vi "HFRR ADV v039 new software.vi"() -> ()   [LabVIEW 2025] (continued)
            n257 = Format Into String(format string="%<%I_%M_%S_%p_%d_%B_%Y>T", w342) -> (resulting string=w341:string)  [unwired: 2 in, 1 out]
            n258 = local write "FILE"(w341) -> ()
          }
        }
        n259 = local read "Auto"() -> (w339:bool)
        n260 = Not(x=w339) -> (.not. x?=w338:bool)
        n261 = local write "Auto"(w338) -> ()
      }
      event "Auto Start Temp": Value Change {
        n262 = event-data() -> ()  [unwired: 1 in, 6 out]
        n263 = local read "Auto Start Test"() -> (w345:bool)
        n264 = case shown="True" w345 {
          frame False {
            n265 = stacked-sequence {
              frame #0 {
                n266 = local write "START TEMP"(FALSE ("START TEMP")) -> ()
              }
              frame #1 {
                n267 = Wait (ms)(milliseconds to wait=u32 2000) -> ()  [unwired: 1 out]
              }
              frame #2 {
                n268 = local write "Due Write"("VC;0") -> ()
              }
              frame #3 {
                n269 = Wait (ms)(milliseconds to wait=u32 2000) -> ()  [unwired: 1 out]
              }
              frame #4 {
                w355 = T19."Enabled" ("Disabled")
                (unwired) T26."Imaging" ("Main Dashboard Buttons")
                w356 = "" ("FILE")
                n270 = local write "Main Tab"(T2."Adv Scar" ("Main Tab")) -> ()
                n271 = local write "measured_stroke"(0.0 ("measured_stroke")) -> ()
                n272 = local write "Main Dashboard Buttons"(T1."Imaging" ("Main Dashboard Buttons")) -> ()
                n273 = property on="RUN" class="Bool (strict)"("Visible"=TRUE) -> ()  [unwired: 2 in, 2 out]
                n274 = local write "Due Write"("VC;0") -> ()
                n275 = local write "TEST FILE NAM,E SAVED"(FALSE ("TEST FILE NAM,E SAVED")) -> ()
                n276 = local write "Fuel Discription :"(w356) -> ()
                n277 = local write "Batch Ref Num :"(w356) -> ()
                n278 = local write "Remarks :"(w356) -> ()
                n279 = local write "FILE"(w356) -> ()
                n280 = property on="FRICVALZ 4" class="Bool (strict)"("DisabledEnum"=w355) -> ()  [unwired: 2 in, 2 out]
                n281 = property on="FRICVALZ 2" class="Bool (strict)"("DisabledEnum"=w355) -> ()  [unwired: 2 in, 2 out]
                n282 = property on="FRICVALZ 3" class="Bool (strict)"("DisabledEnum"=w355) -> ()  [unwired: 2 in, 2 out]
              }
            }
          }
          frame True {
            n283 = stacked-sequence {
              frame #0 {
                n284 = local write "Due Write"("DAC;200") -> ()
              }
              frame #1 {
                n285 = Wait (ms)(milliseconds to wait=u32 1500) -> ()  [unwired: 1 out]
              }
              frame #2 {
                n286 = local write "Due Write"("DAC;200") -> ()
              }
              frame #3 {
                n287 = Wait (ms)(milliseconds to wait=u32 1000) -> ()  [unwired: 1 out]
              }
              frame #4 {
                n288 = local write "Due Write"("VC;1") -> ()
              }
              frame #5 {
                n289 = Wait (ms)(milliseconds to wait=u32 2000) -> ()  [unwired: 1 out]
              }
              frame #6 {
                n290 = local write "Due Write"("VC;1") -> ()
              }
              frame #7 {
                n291 = Wait (ms)(milliseconds to wait=u32 2000) -> ()  [unwired: 1 out]
              }
              frame #8 {
                w367 = T19."Disabled" ("Disabled")
                n292 = property on="RUN" class="Bool (strict)"("Visible"=FALSE) -> ()  [unwired: 2 in, 2 out]
                n293 = property on="FRICVALZ 4" class="Bool (strict)"("DisabledEnum"=w367) -> ()  [unwired: 2 in, 2 out]
                n294 = property on="FRICVALZ 2" class="Bool (strict)"("DisabledEnum"=w367) -> ()  [unwired: 2 in, 2 out]
                n295 = property on="FRICVALZ 3" class="Bool (strict)"("DisabledEnum"=w367) -> ()  [unwired: 2 in, 2 out]
                "START TEMP" <- TRUE
              }
            }
          }
        }
      }
      event "FILE", "USERNAME", "USER ID": Mouse Enter {
        n296 = event-data() -> ()  [unwired: 1 in, 4 out]
        n297 = dll-call lib="kernel32.dll" fn="Wow64DisableWow64FsRedirection"("OldValue"=0) -> (error out=w374:errorcluster, "OldValue"=w372:i32)  [unwired: 4 in, 1 out]
        n298 = call <vilib>:"System Exec.vi"("run minimized? (F)"=TRUE, "error in (no error)"=w374, "command line"="C:\\Program Files\\Common Files\\Microsoft Shared\\Ink\\TabTip.exe") -> ("error out"=w373:errorcluster)  [unwired: 5 in, 3 out]
        n299 = dll-call lib="kernel32.dll" fn="Wow64EnableWow64FsRedirection"(error in=w373, "OldValue"=w372) -> ()  [unwired: 4 in, 2 out]
      }
      event "EDIT": Value Change {
        n300 = event-data() -> ()  [unwired: 1 in, 6 out]
        n301 = local read "EDIT"() -> (w375:bool)
        n302 = case shown="False" w375 {
          frame False {
            n303 = control-ref of="This VI"() -> (w392:refnum<vi>)
            n304 = property class="VI"(reference=w392) -> (reference out=w383:refnum<vi>, error out=w387:errorcluster, "Panel"=w391:refnum<vi>)  [unwired: 1 in]
            n305 = property class="Pnl"(reference=w391, error in=w387) -> (reference out=w385:refnum<vi>, error out=w388:errorcluster, "Panes[]"=w390:refnum<vi>[])
            n306 = for {
              tunnel: w390 -> [w398] mode=indexing
              tunnel: T24."Always Off" ("Horizontal Scrollbar Visibility") -> [w397]
              tunnel: w388 -> [w394]
              tunnel: [w393] -> w386
              n307 = property class="Pane"(reference=w398, error in=w394, "HorizScrollbarVisibility"=w397) -> (reference out=w395:refnum<vi>, error out=w396:errorcluster)
              n308 = Close Reference(reference=w395, error in (no error)=w396) -> (error out=w393:errorcluster)
            }
            n309 = Close Reference(reference=w385, error in (no error)=w386) -> (error out=w384:errorcluster)
            n310 = Close Reference(reference=w383, error in (no error)=w384) -> (error out=w378:errorcluster)
            "error out 7" <- w378
            n311 = call <vilib>:"Clear Errors.vi"("error in (no error)"=w378) -> ("error out"=w377:errorcluster)  [unwired: 5 in, 1 out]
            n312 = local write "Service Password enable"(FALSE ("Service Password enable")) -> ()
            n313 = call <userlib>:"Fit VI window to Largest Dec.vi"("error in (no error)"=w377, "border spacing (2 px)"=1) -> ("error out"=w382:errorcluster, "dup VI Ref"=w380:refnum<vi>)  [unwired: 4 in]
            n314 = invoke on="Invoke Node" class="VI" method="FP.Run-Time Position.Maximized"(reference=w380, error in=w382) -> (error out=w381:errorcluster)  [unwired: 2 in, 3 out]
            n315 = call <vilib>:"Clear Errors.vi"("error in (no error)"=w381) -> ()  [unwired: 5 in, 2 out]
          }
          frame True {
          }
        }
      }
      event "Heater Button": Value Change {
        n316 = event-data() -> ()  [unwired: 1 in, 6 out]
        n317 = local read "Heater Button"() -> (w399:bool)
        n318 = case shown="True" w399 {
          frame True {
            n319 = stacked-sequence {
              frame #0 {
                n320 = Wait (ms)(milliseconds to wait=u32 1500) -> ()  [unwired: 1 out]
              }
              frame #1 {
                n321 = local read "Set Temp"() -> (w401:dbl)
                n322 = Number To Fractional String(number=w401, precision (6)=i16 2) -> (F-format string=w404:string)  [unwired: 2 in]
                n323 = Concatenate Strings("ST;" ("Command"), w404) -> (w403:string)
                n324 = local write "Due Write"(w403) -> ()
              }
              frame #2 {
                n325 = Wait (ms)(milliseconds to wait=u32 1500) -> ()  [unwired: 1 out]
              }
              frame #3 {
                n326 = local write "Due Write"("HE;1" ("Command")) -> ()
              }
              frame #4 {
                n327 = Wait (ms)(milliseconds to wait=u32 1500) -> ()  [unwired: 1 out]
              }
              frame #5 {
                n328 = stacked-sequence {
                  frame #0 {
                    n329 = Wait (ms)(milliseconds to wait=u32 1500) -> ()  [unwired: 1 out]
                  }
                  frame #1 {
                    n330 = local read "Set Temp"() -> (w410:dbl)
                    n331 = Number To Fractional String(number=w410, precision (6)=i16 2) -> (F-format string=w413:string)  [unwired: 2 in]
                    n332 = Concatenate Strings("ST;" ("Command"), w413) -> (w412:string)
                    n333 = local write "Due Write"(w412) -> ()
                  }
                  frame #2 {
                    n334 = Wait (ms)(milliseconds to wait=u32 1500) -> ()  [unwired: 1 out]
                  }
                  frame #3 {
                    n335 = local write "Due Write"("HE;1" ("Command")) -> ()
                  }
                  frame #4 {
                    n336 = Wait (ms)(milliseconds to wait=u32 1500) -> ()  [unwired: 1 out]
                  }
                }
              }
            }
          }
          frame False {
            n337 = stacked-sequence {
              frame #0 {
                n338 = Wait (ms)(milliseconds to wait=u32 1500) -> ()  [unwired: 1 out]
              }
              frame #1 {
                n339 = Concatenate Strings("ST;" ("Command"), "0" ("string")) -> (w420:string)
                n340 = local write "Due Write"(w420) -> ()
              }
              frame #2 {
                n341 = Wait (ms)(milliseconds to wait=u32 1500) -> ()  [unwired: 1 out]
              }
              frame #3 {
                n342 = local write "Due Write"("HE;0" ("Command")) -> ()
              }
              frame #4 {
                n343 = Wait (ms)(milliseconds to wait=u32 1500) -> ()  [unwired: 1 out]
              }
            }
          }
        }
      }
      event "Headen Service Button": Value Change {
        n344 = event-data() -> ()  [unwired: 1 in, 6 out]
        n345 = local read "Headen Service Button"() -> (w425:bool)
        n346 = case shown="True" w425 {
          frame False {
            n347 = property on="Password 3" class="Clust (strict)"("Visible"=FALSE) -> ()  [unwired: 2 in, 2 out]
            n348 = property on="Service Password Log" class="Str"("Visible"=FALSE) -> ()  [unwired: 2 in, 2 out]
          }
          frame True {
            n349 = property on="Password 3" class="Clust (strict)"("Visible"=TRUE) -> ()  [unwired: 2 in, 2 out]
            n350 = property on="Service Password Log" class="Str"("Visible"=TRUE) -> ()  [unwired: 2 in, 2 out]
          }
        }
      }
      event "Password 3.Service Password": Value Change {
        n351 = event-data() -> ()  [unwired: 1 in, 6 out]
        n352 = Unbundle By Name("Password 3") -> ("Service Password"=w432:string)
        n353 = call <vilib>:"Trim Whitespace.vi"("string"=w432) -> ("trimmed string"=w430:string)  [unwired: 1 in]
        n354 = Equal?(x=w430, y="Service@123") -> (x = y?=w431:bool)
        n355 = case shown="False" w431 {
          selector: w431 -> [w435 w437]
          frame False {
            n356 = local write "Service Password enable"(w435) -> ()
            n357 = property on="Service Password Log" class="Str"("Visible"=TRUE) -> ()  [unwired: 2 in, 2 out]
          }
          frame True {
            n358 = property on="Service Password Log" class="Str"("Visible"=FALSE) -> ()  [unwired: 2 in, 2 out]
            "Service Password enable" <- w437
          }
        }
      }
      event "Sign In": Value Change {
        w439 = FALSE ("Visible")
        n359 = event-data() -> ()  [unwired: 1 in, 6 out]
        n360 = property on="About" class="Clust (strict)"("Visible"=w439) -> ()  [unwired: 2 in, 2 out]
        n361 = property on="Password 3" class="Clust (strict)"("Visible"=w439) -> ()  [unwired: 2 in, 2 out]
        n362 = property on="Service Password Log" class="Str"("Visible"=FALSE) -> ()  [unwired: 2 in, 2 out]
      }
      event "Info": Value Change {
        n363 = event-data() -> ()  [unwired: 1 in, 6 out]
        n364 = local read "Info"() -> (w441:bool)
        n365 = case shown="False" w441 {
          frame False {
            n366 = property on="About" class="Clust (strict)"("Visible"=FALSE) -> ()  [unwired: 2 in, 2 out]
          }
          frame True {
            n367 = property on="About" class="Clust (strict)"("Visible"=TRUE) -> ()  [unwired: 2 in, 2 out]
          }
        }
      }
      event "Calibration": Value Change {
        n368 = event-data() -> ()  [unwired: 1 in, 6 out]
        n369 = local read "Calibration"() -> (w445:bool)
        n370 = case shown="False" w445 {
          frame False {
            n371 = local write "Cal Password"("" ("Cal Password")) -> ()
            n372 = property on="Calibration 2" class="TabCtl (strict)"("Visible"=FALSE) -> ()  [unwired: 2 in, 2 out]
          }
          frame True {
            n373 = property on="Calibration 2" class="TabCtl (strict)"("Visible"=TRUE) -> ()  [unwired: 2 in, 2 out]
            n374 = local write "Cal Password"("" ("Cal Password")) -> ()
          }
        }
        n375 = property on="Wrong Password" class="Str"("Visible"=FALSE) -> ()  [unwired: 2 in, 2 out]
      }
      event "Cal Password": Value Change {
        n376 = event-data() -> ()  [unwired: 1 in, 6 out]
        n377 = local read "Cal Password"() -> (w453:string)
        n378 = call <vilib>:"Trim Whitespace.vi"("string"=w453) -> ("trimmed string"=w452:string)  [unwired: 1 in]
        n379 = Equal?(x=w452, y="Cal@321") -> (x = y?=w450:bool)
        n380 = case shown="True" w450 {
          frame False {
            n381 = property on="Wrong Password" class="Str"("Visible"=TRUE) -> ()  [unwired: 2 in, 2 out]
          }
          frame True {
            n382 = property on="Wrong Password" class="Str"("Visible"=FALSE) -> ()  [unwired: 2 in, 2 out]
            n383 = local write "Main Tab"(T2."About" ("Main Tab")) -> ()
            n384 = local write "Cal Password"("" ("Cal Password")) -> ()
            n385 = local write "Main Dashboard Buttons"(T1."About" ("Main Dashboard Buttons")) -> ()
            n386 = property on="Calibration 2" class="TabCtl (strict)"("Visible"=FALSE) -> ()  [unwired: 2 in, 2 out]
            n387 = local write "Calibration"(FALSE ("Calibration")) -> ()
          }
        }
      }
      event "Calibration Selection": Value Change {
        n388 = event-data() -> ()  [unwired: 1 in, 6 out]
        n389 = local read "Calibration Selection"() -> (w462:T8)
        n390 = case shown="\"Stroke Calibration\"" w462 {
          tunnel: [T7."Stroke" ("Main Calibration Tab") T7."Friction" ("Main Calibration Tab") T7."Main" ("Main Calibration Tab") T7."Temperature" ("Main Calibration Tab")] -> w461
          frame "Stroke Calibration" {
          }
          frame "Friction Force Calibration" {
          }
          frame Default {
          }
          frame "Temperature Calibration" {
          }
        }
        n391 = local write "Main Calibration Tab"(w461) -> ()
      }
      event "Back Stroke": Value Change {
        n392 = event-data() -> ()  [unwired: 1 in, 6 out]
        n393 = local write "Main Stroke Tab"(T9."Step 1" ("Main Stroke Tab")) -> ()
        n394 = local write "Main Calibration Tab"(T7."Main" ("Main Calibration Tab")) -> ()
        n395 = local write "Back Stroke"(FALSE ("Back Stroke")) -> ()
      }
      event "Step 2 Back": Value Change {
        n396 = event-data() -> ()  [unwired: 1 in, 6 out]
        n397 = local write "Main Stroke Tab"(T9."Step 1" ("Main Stroke Tab")) -> ()
        n398 = local write "Step 2 Back"(FALSE ("Back Stroke")) -> ()
      }
      event "Step 3 Back": Value Change {
        n399 = event-data() -> ()  [unwired: 1 in, 6 out]
        n400 = local write "Main Stroke Tab"(T9."Step 2" ("Main Stroke Tab")) -> ()
        n401 = local write "Step 3 Back"(FALSE ("Back Stroke")) -> ()
      }
      event "Step 4 Back": Value Change {
        n402 = event-data() -> ()  [unwired: 1 in, 6 out]
        n403 = local write "Main Stroke Tab"(T9."Step 3" ("Main Stroke Tab")) -> ()
        n404 = local write "Step 4 Back"(FALSE ("Back Stroke")) -> ()
      }
      event "Step 5 Back": Value Change {
        n405 = event-data() -> ()  [unwired: 1 in, 6 out]
        n406 = local write "Main Stroke Tab"(T9."Step 4" ("Main Stroke Tab")) -> ()
        n407 = local write "Step 5 Back"(FALSE ("Back Stroke")) -> ()
      }
      event "Step 6 Back": Value Change {
        n408 = event-data() -> ()  [unwired: 1 in, 6 out]
        n409 = local write "Main Stroke Tab"(T9."Step 5" ("Main Stroke Tab")) -> ()
        n410 = local write "Step 6 Back"(FALSE ("Back Stroke")) -> ()
      }
      event "Back Stroke step 7": Value Change {
        n411 = event-data() -> ()  [unwired: 1 in, 6 out]
        n412 = local write "Main Stroke Tab"(T9."Step 5" ("Main Stroke Tab")) -> ()
        n413 = local write "Back Stroke step 7"(FALSE ("Back Stroke")) -> ()
      }
      event "Back Stroke step 8": Value Change {
        n414 = event-data() -> ()  [unwired: 1 in, 6 out]
        n415 = local write "Main Stroke Tab"(T9."Step 7" ("Main Stroke Tab")) -> ()
        n416 = local write "Back Stroke step 8"(FALSE ("Back Stroke")) -> ()
      }
      event "Back Stroke 8": Value Change {
        n417 = event-data() -> ()  [unwired: 1 in, 6 out]
        n418 = local write "MOVE CARRIAGE TO"(0.2 ("MOVE CARRIAGE TO")) -> ()
        n419 = local write "Main Stroke Tab"(T9."Step 1" ("Main Stroke Tab")) -> ()
        n420 = local write "Back Stroke 8"(FALSE ("Back Stroke 8")) -> ()
      }
      event "Continue Stroke": Value Change {
        n421 = event-data() -> ()  [unwired: 1 in, 6 out]
        n422 = local write "Main Stroke Tab"(T9."Step 2" ("Main Stroke Tab")) -> ()
        n423 = local write "Continue Stroke"(FALSE ("Continue Stroke")) -> ()
      }
      event "Continue Stroke step 2": Value Change {
        n424 = event-data() -> ()  [unwired: 1 in, 6 out]
        n425 = local write "Main Stroke Tab"(T9."Step 3" ("Main Stroke Tab")) -> ()
        n426 = local write "Continue Stroke step 2"(FALSE ("Continue Stroke")) -> ()
      }
      event "Continue Stroke step 3": Value Change {
        n427 = event-data() -> ()  [unwired: 1 in, 6 out]
        n428 = local write "Main Stroke Tab"(T9."Step 4" ("Main Stroke Tab")) -> ()
        n429 = local write "Continue Stroke step 3"(FALSE ("Continue Stroke")) -> ()
      }
      event "Continue Stroke step 4": Value Change {
        n430 = event-data() -> ()  [unwired: 1 in, 6 out]
        n431 = local write "Main Stroke Tab"(T9."Step 5" ("Main Stroke Tab")) -> ()
        n432 = local write "Continue Stroke step 4"(FALSE ("Continue Stroke")) -> ()
      }
      event "Continue Stroke step 5": Value Change {
        n433 = event-data() -> ()  [unwired: 1 in, 6 out]
        n434 = local write "Main Stroke Tab"(T9."Step 7" ("Main Stroke Tab")) -> ()
        n435 = local write "Continue Stroke step 5"(FALSE ("Continue Stroke")) -> ()
      }
      event "Continue Stroke step 6": Value Change {
        n436 = event-data() -> ()  [unwired: 1 in, 6 out]
        n437 = local write "Main Stroke Tab"(T9."Step 7" ("Main Stroke Tab")) -> ()
        n438 = local write "Continue Stroke step 6"(FALSE ("Continue Stroke")) -> ()
      }
      event "Continue Stroke step 7": Value Change {
        w501 = FALSE ("0.2mm")
        n439 = event-data() -> ()  [unwired: 1 in, 6 out]
        n440 = local write "1.2"(w501) -> ()
        n441 = local write "1.0 2"(w501) -> ()
        n442 = local write "0.8 2"(w501) -> ()
        n443 = local write "0.6 2"(w501) -> ()
        n444 = local write "0.4 2"(w501) -> ()
        n445 = local write "0.2 2"(w501) -> ()
        n446 = local write "1.2 mm"(w501) -> ()
        n447 = local write "1.0 mm"(w501) -> ()
        n448 = local write "0.6 mm"(w501) -> ()
        n449 = local write "0.4 mm"(w501) -> ()
        n450 = local write "0.8mm"(w501) -> ()
        n451 = local write "0.2mm"(w501) -> ()
        n452 = local write "Main Stroke Tab"(T9."Step 8" ("Main Stroke Tab")) -> ()
        n453 = local write "Continue Stroke step 7"(FALSE ("Continue Stroke")) -> ()
        n454 = local write "Stroke Test Complete"(T10."Test Progress" ("Stroke Test Complete")) -> ()
        "Position Measurment Temp" <- 4.0 ("Position Measurment Temp")
        "Calibration Tare" <- TRUE ("Calibration Tare")
        "MOVE CARRIAGE TO" <- 1.0 ("MOVE CARRIAGE TO")
      }
      event "Continue Stroke step 8": Value Change {
        n455 = event-data() -> ()  [unwired: 1 in, 6 out]
        n456 = local read "LVDT STROKE  Calibration"() -> (w506:dbl)
        n457 = local read "Position Measurment Temp"() -> (w507:dbl)
        n458 = case shown="7" w507 {
          selector: w507 -> [_ w512 w520 w525 _ w533 w536 w537]
          tunnel: w506 -> [w509 w513 w516 w521 w527 w530 _ _]
          frame 0, Default {
            w511 = TRUE ("0.2mm")
            n459 = local write "Position Measurment Temp"(4.0 ("Position Measurment Temp")) -> ()
            n460 = local write "0.2mm"(w511) -> ()
            n461 = local write "0.2 2"(w511) -> ()
            n462 = local write "MOVE CARRIAGE TO"(1.0 ("MOVE CARRIAGE TO")) -> ()
            "Calibration 0.2" <- w509
          }
          frame 1 {
            w515 = TRUE ("0.4 mm")
            n463 = local write "Calibration 0.4"(w513) -> ()
            n464 = local write "Position Measurment Temp"(w512) -> ()
            n465 = local write "0.4 mm"(w515) -> ()
            n466 = local write "MOVE CARRIAGE TO"(0.6 ("MOVE CARRIAGE TO")) -> ()
            n467 = local write "0.4 2"(w515) -> ()
          }
          frame 2 {
            w518 = TRUE ("0.6 mm")
            n468 = Increment(x=w520) -> (x+1=w519:i32)
            n469 = local write "Calibration 0.6"(w516) -> ()
            n470 = local write "Position Measurment Temp"(w519) -> ()
            n471 = local write "0.6 2"(w518) -> ()
            n472 = local write "0.6 mm"(w518) -> ()
            n473 = local write "MOVE CARRIAGE TO"(0.8 ("MOVE CARRIAGE TO")) -> ()
          }
          frame 3 {
            w522 = TRUE ("0.6 mm")
            n474 = Increment(x=w525) -> (x+1=w524:i32)
            n475 = local write "Position Measurment Temp"(w524) -> ()
            n476 = local write "MOVE CARRIAGE TO"(1.0 ("MOVE CARRIAGE TO")) -> ()
            n477 = local write "0.8mm"(w522) -> ()
            n478 = local write "0.8 2"(w522) -> ()
            "Calibration 0.8" <- w521
          }
          frame 4 {
            w528 = TRUE ("0.6 mm")
            n479 = local write "Position Measurment Temp"(6.0 ("Position Measurment Temp")) -> ()
            n480 = local write "MOVE CARRIAGE TO"(1.0 ("MOVE CARRIAGE TO")) -> ()
            n481 = local write "1.0 mm"(w528) -> ()
            n482 = local write "1.0 2"(w528) -> ()
            "Calibration 1.0" <- w527
          }
          frame 5 {
            w531 = TRUE ("0.6 mm")
            n483 = Increment(x=w533) -> (x+1=w532:i32)
            n484 = local write "Position Measurment Temp"(w532) -> ()
            n485 = local write "1.2 mm"(w531) -> ()
            n486 = local write "1.2"(w531) -> ()
            "Calibration 1.2" <- w530
          }
          frame 6 {
            n487 = Increment(x=w536) -> (x+1=w535:i32)
            n488 = local write "Position Measurment Temp"(w535) -> ()
            n489 = local write "Stroke Test Complete"(T10."Stroke Points Completed" ("Stroke Test Complete")) -> ()
          }
          frame 7 {
            n490 = stacked-sequence {
              tunnel: w537 -> [w538 _ _]
              frame #0 {
                n491 = Increment(x=w538) -> (x+1=w539:i32)
                n492 = local write "Main Stroke Tab"(T9."Step 9" ("Main Stroke Tab")) -> ()
                n493 = local write "Position Measurment Temp"(w539) -> ()
                n494 = Insert Into Array(array=dbl[] [], new element #1=0.2 ("new element/subarray"), new element #2=0.4 ("new element/subarray"), new element #3=0.6 ("new element/subarray"), new element #4=0.8 ("new element/subarray"), new element #5=1.0 ("new element/subarray"), new element #6=1.2 ("new element/subarray")) -> (→"1D stroke":dbl[])  [unwired: 1 in]
                n495 = local read "Calibration 1.2"() -> (w541:dbl)
                n496 = local read "Calibration 1.0"() -> (w542:dbl)
                n497 = local read "Calibration 0.8"() -> (w543:dbl)
                n498 = local read "Calibration 0.6"() -> (w544:dbl)
                n499 = local read "Calibration 0.4"() -> (w545:dbl)
                n500 = local read "Calibration 0.2"() -> (w546:dbl)
                n501 = Insert Into Array(array=dbl[] [], new element #1=w546, new element #2=w545, new element #3=w544, new element #4=w543, new element #5=w542, new element #6=w541) -> (→"Calibrated Voltage Value":dbl[])  [unwired: 1 in]
              }
              frame #1 {
                n502 = local read "calibration values"() -> (w569:dbl[])
                n503 = local read "Calibrated Voltage Value"() -> (w571:dbl[])
                n504 = Index Array(array=w569, index #1=1 ("index"), index #2=3 ("index"), index #3=5 ("index"), index #4=7 ("index"), index #5=9 ("index"), index #6=11 ("index")) -> (element #1=w562:dbl, element #2=w561:dbl, element #3=w560:dbl, element #4=w559:dbl, element #5=w558:dbl, element #6=w557:dbl)
                n505 = local read "1D stroke"() -> (w572:dbl[])
                n506 = for {
                  tunnel: [w581] -> w570 mode=indexing
                  tunnel: w572 -> [w580] mode=indexing
                  tunnel: w571 -> [w579] mode=indexing
                  tunnel: w562 -> [w578]
                  tunnel: w561 -> [w577]
                  tunnel: w560 -> [w576]
                  tunnel: w559 -> [w575]
                  tunnel: w558 -> [w574]
                  tunnel: w557 -> [w573]
                  n507 = formula code="if (stroke == 0.2)\n{\n    if ((voltage >= REF_02 - 0.2) && (voltage <= REF_02 + 0.2))\n        status = 1;\n    else\n        status = 0;\n}\nelse if (stroke == 0.4)\n{\n    if ((voltage >= REF_04 - 0.2) && (voltage <= REF_04 + 0.2))\n        status = 1;\n    else\n        status = 0;\n}\nelse if (stroke == 0.6)\n{\n    if ((voltage >= REF_06 - 0.2) && (voltage <= REF_06 + 0.2))\n        status = 1;\n    else\n        status = 0;\n}\nelse if (stroke == 0.8)\n{\n    if ((voltage >= REF_08 - 0.2) && (voltage <= REF_08 + 0.2))\n        status = 1;\n    else\n        status = 0;\n}\nelse if (stroke == 1.0)\n{\n    if ((voltage >= REF_10 - 0.6) && (voltage <= REF_10 + 0.6))\n        status = 1;\n    else\n        status = 0;\n}\nelse if (stroke == 1.2)\n{\n    if ((voltage >= REF_12 - 0.2) && (voltage <= REF_12 + 0.2))\n        status = 1;\n    else\n        status = 0;\n}\nelse\n{\n    status = 0;\n}"("stroke"=w580, "voltage"=w579, "REF_02"=w578, "REF_04"=w577, "REF_06"=w576, "REF_08"=w575, "REF_10"=w574, "REF_12"=w573) -> ("status"=w581:dbl)
                }
                "Status" <- w570
              }
              frame #2 {
                w588 = 1.0
                n508 = local read "Status"() -> (w595:dbl[])
                n509 = Index Array(array=w595) -> (element #1=w594:dbl, element #2=w593:dbl, element #3=w592:dbl, element #4=w591:dbl, element #5=w590:dbl, element #6=w589:dbl)  [unwired: 6 in]
                n510 = Equal?(x=w589, y=w588) -> (x = y?=w582:bool)
                n511 = Equal?(x=w590, y=w588) -> (x = y?=w583:bool)
                n512 = Equal?(x=w591, y=w588) -> (x = y?=w584:bool)
                n513 = Equal?(x=w592, y=w588) -> (x = y?=w585:bool)
                n514 = Equal?(x=w593, y=w588) -> (x = y?=w586:bool)
                n515 = Equal?(x=w594, y=w588) -> (x = y?=w587:bool)
                n516 = case shown="True" w587 {
                  selector: w587 -> [w606 w607]
                  frame True {
                    n517 = local write "Point 1 - 0.2 mm"(w606) -> ()
                    n518 = property on="Point 1 - 0.2 mm" class="Bool"("Caption.Visible"=w606) -> ()  [unwired: 2 in, 2 out]
                  }
                  frame False {
                    n519 = local write "Point 1 - 0.2 mm"(w607) -> ()
                    n520 = property on="Point 1 - 0.2 mm" class="Bool"("Caption.Visible"=w607) -> ()  [unwired: 2 in, 2 out]
                  }
                }
                n521 = case shown="True" w583 {
                  selector: w583 -> [w598 w599]
                  frame True {
                    n522 = local write "Point 5 - 1.0 mm"(w598) -> ()
                    n523 = property on="Point 5 - 1.0 mm" class="Bool"("Caption.Visible"=w598) -> ()  [unwired: 2 in, 2 out]
                  }
                  frame False {
                    n524 = local write "Point 5 - 1.0 mm"(w599) -> ()
                    n525 = property on="Point 5 - 1.0 mm" class="Bool"("Caption.Visible"=w599) -> ()  [unwired: 2 in, 2 out]
                  }
                }
                n526 = case shown="True" w586 {
                  selector: w586 -> [w604 w605]
                  frame True {
                    n527 = local write "Point 2 - 0.4 mm"(w604) -> ()
                    n528 = property on="Point 2 - 0.4 mm" class="Bool"("Caption.Visible"=w604) -> ()  [unwired: 2 in, 2 out]
                  }
                  frame False {
                    n529 = local write "Point 2 - 0.4 mm"(w605) -> ()
                    n530 = property on="Point 2 - 0.4 mm" class="Bool"("Caption.Visible"=w605) -> ()  [unwired: 2 in, 2 out]
                  }
                }
                n531 = case shown="True" w582 {
                  selector: w582 -> [w596 w597]
                  frame True {
                    n532 = local write "Point 6 - 1.2 mm"(w596) -> ()
                    n533 = property on="Point 6 - 1.2 mm" class="Bool"("Caption.Visible"=w596) -> ()  [unwired: 2 in, 2 out]
                  }
                  frame False {
                    n534 = local write "Point 6 - 1.2 mm"(w597) -> ()
                    n535 = property on="Point 6 - 1.2 mm" class="Bool"("Caption.Visible"=w597) -> ()  [unwired: 2 in, 2 out]
                  }
                }
                n536 = case shown="True" w584 {
                  selector: w584 -> [w600 w601]
                  frame True {
                    n537 = local write "Point 4 - 0.8 mm"(w600) -> ()
                    n538 = property on="Point 4 - 0.8 mm" class="Bool"("Caption.Visible"=w600) -> ()  [unwired: 2 in, 2 out]
                  }
                  frame False {
                    n539 = local write "Point 4 - 0.8 mm"(w601) -> ()
                    n540 = property on="Point 4 - 0.8 mm" class="Bool"("Caption.Visible"=w601) -> ()  [unwired: 2 in, 2 out]
                  }
                }
                n541 = case shown="True" w585 {
                  selector: w585 -> [w602 w603]
                  frame True {
                    n542 = local write "Point 3 - 0.6 mm"(w602) -> ()
                    n543 = property on="Point 3 - 0.6 mm" class="Bool"("Caption.Visible"=w602) -> ()  [unwired: 2 in, 2 out]
                  }
                  frame False {
                    n544 = local write "Point 3 - 0.6 mm"(w603) -> ()
                    n545 = property on="Point 3 - 0.6 mm" class="Bool"("Caption.Visible"=w603) -> ()  [unwired: 2 in, 2 out]
                  }
                }
              }
            }
          }
        }
      }
      event "TEMPERATURE STEP Back 1", "TEMPERATURE STEP Back air Temp": Value Change {
        n546 = event-data() -> ()  [unwired: 1 in, 6 out]
        n547 = stacked-sequence {
          frame #0 {
            n548 = local write "Main Calibration Tab"(T7."Main" ("Main Calibration Tab")) -> ()
          }
          frame #1 {
            n549 = Wait (ms)(milliseconds to wait=u32 1000) -> ()  [unwired: 1 out]
          }
          frame #2 {
            n550 = local write "Due Write"("CAL;END" ("Command")) -> ()
          }
          frame #3 {
            n551 = Wait (ms)(milliseconds to wait=u32 2000) -> ()  [unwired: 1 out]
          }
          frame #4 {
            n552 = local write "Due Write"("CAL;END" ("Command")) -> ()
          }
        }
      }
      event "Temperature Continue Step 1": Value Change {
        n553 = event-data() -> ()  [unwired: 1 in, 6 out]
        n554 = stacked-sequence {
          frame #0 {
            n555 = Wait (ms)(milliseconds to wait=u32 1500) -> ()  [unwired: 1 out]
          }
          frame #1 {
            n556 = local write "Due Write"("CAL;START" ("Command")) -> ()
          }
          frame #2 {
            n557 = Wait (ms)(milliseconds to wait=u32 1500) -> ()  [unwired: 1 out]
          }
          frame #3 {
            n558 = local write "Due Write"("CAL;START" ("Command")) -> ()
          }
          frame #4 {
            n559 = Wait (ms)(milliseconds to wait=u32 2000) -> ()  [unwired: 1 out]
          }
          frame #5 {
          }
          frame #6 {
            n560 = Wait (ms)(milliseconds to wait=u32 2000) -> ()  [unwired: 1 out]
          }
          frame #7 {
            # "CAL;A1;<true_T>"
            n561 = local write "Due Write"("CAL;A1;0" ("Command")) -> ()
          }
          frame #8 {
            n562 = local write "Tab Control 4"(T12."Step 2" ("Tab Control 4")) -> ()
          }
        }
      }
      event "Temperature Continue Step air Step 1": Value Change {
        n563 = event-data() -> ()  [unwired: 1 in, 6 out]
        n564 = stacked-sequence {
          frame #0 {
            n565 = Wait (ms)(milliseconds to wait=u32 1500) -> ()  [unwired: 1 out]
          }
          frame #1 {
            n566 = local write "Due Write"("CAL;START" ("Command")) -> ()
          }
          frame #2 {
            n567 = Wait (ms)(milliseconds to wait=u32 1500) -> ()  [unwired: 1 out]
          }
          frame #3 {
            n568 = local write "Due Write"("CAL;START" ("Command")) -> ()
          }
          frame #4 {
          }
          frame #5 {
          }
          frame #6 {
            n569 = Wait (ms)(milliseconds to wait=u32 2000) -> ()  [unwired: 1 out]
          }
          frame #7 {
            # "CAL;A1;<true_T>"
            n570 = local write "Due Write"("CAL;A1;0" ("Command")) -> ()
          }
          frame #8 {
            n571 = local write "Tab Control 4"(T12."Air Step 2" ("Tab Control 4")) -> ()
          }
        }
      }
      event "Temperature Selection": Value Change {
        n572 = event-data() -> ()  [unwired: 1 in, 6 out]
        n573 = local read "Temperature Selection"() -> (w628:T13)
        n574 = case shown="\"Default\", Default" w628 {
          frame "Air Temperature" {
            n575 = local write "Tab Control 4"(T12."Air Step 1" ("Tab Control 4")) -> ()
          }
          frame "Sample Temperature" {
            n576 = local write "Tab Control 4"(T12."Step 1" ("Tab Control 4")) -> ()
          }
          frame "Default", Default {
          }
        }
      }
      event "Temperature Continue Step 2": Value Change {
        n577 = event-data() -> ()  [unwired: 1 in, 6 out]
        n578 = stacked-sequence {
          frame #0 {
            n579 = stacked-sequence {
              frame #0 {
                n580 = Wait (ms)(milliseconds to wait=u32 1500) -> ()  [unwired: 1 out]
              }
              frame #1 {
                # "CAL;A1;<true_T>"
                n581 = local write "Due Write"("CAL;A1;0" ("Command")) -> ()
              }
              frame #2 {
                n582 = Wait (ms)(milliseconds to wait=u32 1500) -> ()  [unwired: 1 out]
              }
              frame #3 {
                # "CAL;A1;<true_T>"
                n583 = local write "Due Write"("CAL;A1;0" ("Command")) -> ()
              }
              frame #4 {
              }
            }
          }
          frame #1 {
            n584 = local read "Sensor value"() -> (→"Sensor value  zero degree sample":dbl)
            n585 = local write "Tab Control 4"(T12."Step 3" ("Tab Control 4")) -> ()
          }
        }
      }
      event "Record Point Air Temp Step 2": Value Change {
        n586 = event-data() -> ()  [unwired: 1 in, 6 out]
        n587 = stacked-sequence {
          frame #0 {
            n588 = stacked-sequence {
              frame #0 {
                n589 = Wait (ms)(milliseconds to wait=u32 1500) -> ()  [unwired: 1 out]
              }
              frame #1 {
                # "CAL;A1;<true_T>"
                n590 = local write "Due Write"("CAL;A1;0" ("Command")) -> ()
              }
              frame #2 {
                n591 = Wait (ms)(milliseconds to wait=u32 1500) -> ()  [unwired: 1 out]
              }
              frame #3 {
                # "CAL;A1;<true_T>"
                n592 = local write "Due Write"("CAL;A1;0" ("Command")) -> ()
              }
              frame #4 {
              }
            }
          }
          frame #1 {
            (unwired) 0.0 ("Sensor value")
            n593 = local read "Sensor value"() -> (→"Air Temp zero ded":dbl)
            n594 = local write "Tab Control 4"(T12."Air Step 3" ("Tab Control 4")) -> ()
          }
        }
      }
      event "Temperature Continue Step 3": Value Change {
        n595 = event-data() -> ()  [unwired: 1 in, 6 out]
        n596 = stacked-sequence {
          frame #0 {
            n597 = stacked-sequence {
              frame #0 {
                n598 = Wait (ms)(milliseconds to wait=u32 1500) -> ()  [unwired: 1 out]
              }
              frame #1 {
              }
              frame #2 {
              }
              frame #3 {
                # "CAL;A1;<true_T>"
                n599 = local write "Due Write"("CAL;A1;60" ("Command")) -> ()
              }
              frame #4 {
                n600 = Wait (ms)(milliseconds to wait=u32 2000) -> ()  [unwired: 1 out]
              }
              frame #5 {
                # "CAL;A1;<true_T>"
                n601 = local write "Due Write"("CAL;A1;60" ("Command")) -> ()
              }
            }
          }
          frame #1 {
          }
          frame #2 {
          }
          frame #3 {
          }
          frame #4 {
          }
          frame #5 {
          }
          frame #6 {
            # "CAL;END"
          }
          frame #7 {
          }
          frame #8 {
            # "CAL;END"
          }
          frame #9 {
            n602 = local read "Sensor value"() -> (→"Sensor value 60 deg sample":dbl)
            n603 = local write "Tab Control 4"(T12."Step 4" ("Tab Control 4")) -> ()
          }
          frame #10 {
            n604 = local read "Sensor value  zero degree sample"() -> (w657:dbl)
            n605 = local read "Sensor value 60 deg sample"() -> (w656:dbl)
            n606 = In Range and Coerce(upper limit=62.0, x=w656, lower limit=58.0) -> (In Range?=w650:bool)  [unwired: 1 out]
            n607 = In Range and Coerce(upper limit=1.0, x=w657, lower limit=-1.0) -> (In Range?=w651:bool)  [unwired: 1 out]
            n608 = And(x=w651, y=w650) -> (x .and. y?=w649:bool)
            n609 = case shown="True" w649 {
              frame False {
                n610 = property on="Accept & Save sample Temperature step 4" class="Bool (strict)"("DisabledEnum"=T19."Disabled" ("Disabled")) -> ()  [unwired: 2 in, 2 out]
                n611 = local write "Sample Temperature Calibration"(enum32{"True", "Fail"}."Fail" ("Sample Temperature Calibration")) -> ()
              }
              frame True {
                n612 = property on="Accept & Save sample Temperature step 4" class="Bool (strict)"("DisabledEnum"=T19."Enabled" ("Disabled")) -> ()  [unwired: 2 in, 2 out]
                n613 = local write "Sample Temperature Calibration"(enum32{"True", "Fail"}."True" ("Sample Temperature Calibration")) -> ()
              }
            }
          }
        }
      }
      event "Accept & Save sample Temperature step 4": Value Change {
        n614 = event-data() -> ()  [unwired: 1 in, 6 out]
        n615 = stacked-sequence {
          frame #0 {
          }
          frame #1 {
            n616 = local write "Due Write"("CAL;SAVE" ("Command")) -> ()
          }
          frame #2 {
            n617 = Wait (ms)(milliseconds to wait=u32 1000) -> ()  [unwired: 1 out]
          }
          frame #3 {
            n618 = local write "Due Write"("CAL;SAVE" ("Command")) -> ()
          }
          frame #4 {
            n619 = Wait (ms)(milliseconds to wait=u32 1000) -> ()  [unwired: 1 out]
          }
          frame #5 {
            n620 = local write "Due Write"("CAL;END" ("Command")) -> ()
          }
          frame #6 {
            n621 = Wait (ms)(milliseconds to wait=u32 1000) -> ()  [unwired: 1 out]
          }
          frame #7 {
            n622 = local write "Due Write"("CAL;END" ("Command")) -> ()
          }
          frame #8 {
            n623 = local write "Main Calibration Tab"(T7."Temperature" ("Main Calibration Tab")) -> ()
            n624 = local write "Tab Control 4"(T12."Main" ("Tab Control 4")) -> ()
          }
        }
      }
      event "Accept & Save sample Temperature step 5": Value Change {
        n625 = event-data() -> ()  [unwired: 1 in, 6 out]
        n626 = stacked-sequence {
          frame #0 {
          }
          frame #1 {
            n627 = local write "Due Write"("CAL;SAVE" ("Command")) -> ()
          }
          frame #2 {
            n628 = Wait (ms)(milliseconds to wait=u32 1000) -> ()  [unwired: 1 out]
          }
          frame #3 {
            n629 = local write "Due Write"("CAL;SAVE" ("Command")) -> ()
          }
          frame #4 {
            n630 = Wait (ms)(milliseconds to wait=u32 1000) -> ()  [unwired: 1 out]
          }
          frame #5 {
            n631 = local write "Due Write"("CAL;END" ("Command")) -> ()
          }
          frame #6 {
            n632 = Wait (ms)(milliseconds to wait=u32 1000) -> ()  [unwired: 1 out]
          }
          frame #7 {
            n633 = local write "Due Write"("CAL;END" ("Command")) -> ()
          }
          frame #8 {
            n634 = local write "Main Calibration Tab"(T7."Temperature" ("Main Calibration Tab")) -> ()
            n635 = local write "Tab Control 4"(T12."Main" ("Tab Control 4")) -> ()
          }
        }
      }
      event "Temperature Continue Step 6": Value Change {
        n636 = event-data() -> ()  [unwired: 1 in, 6 out]
        n637 = stacked-sequence {
          frame #0 {
            n638 = Wait (ms)(milliseconds to wait=u32 1500) -> ()  [unwired: 1 out]
          }
          frame #1 {
            # "CAL;A1;<true_T>"
            n639 = local write "Due Write"("CAL;A1;60" ("Command")) -> ()
          }
          frame #2 {
            n640 = Wait (ms)(milliseconds to wait=u32 2000) -> ()  [unwired: 1 out]
          }
          frame #3 {
            # "CAL;A1;<true_T>"
            n641 = local read "Sensor value"() -> (→"Air Temp 60 deg":dbl)
            n642 = local write "Due Write"("CAL;A1;60" ("Command")) -> ()
          }
          frame #4 {
            n643 = local read "Air Temp zero ded"() -> (w685:dbl)
            n644 = local read "Air Temp 60 deg"() -> (w686:dbl)
            n645 = In Range and Coerce(upper limit=1.0, x=w685, lower limit=-1.0) -> (In Range?=w693:bool)  [unwired: 1 out]
            n646 = In Range and Coerce(upper limit=62.0, x=w686, lower limit=58.0) -> (In Range?=w692:bool)  [unwired: 1 out]
            n647 = And(x=w693, y=w692) -> (x .and. y?=w691:bool)
            n648 = case shown="True" w691 {
              frame False {
                n649 = local write "Sample Temperature Calibration  2"(enum32{"True", "Fail"}."Fail" ("Sample Temperature Calibration")) -> ()
                n650 = property on="Accept & Save sample Temperature step 5" class="Bool (strict)"("DisabledEnum"=T19."Disabled" ("Disabled")) -> ()  [unwired: 2 in, 2 out]
              }
              frame True {
                n651 = local write "Sample Temperature Calibration  2"(enum32{"True", "Fail"}."True" ("Sample Temperature Calibration")) -> ()
                n652 = property on="Accept & Save sample Temperature step 5" class="Bool (strict)"("DisabledEnum"=T19."Enabled" ("Disabled")) -> ()  [unwired: 2 in, 2 out]
              }
            }
          }
          frame #5 {
            n653 = local write "Tab Control 4"(T12."Air Step 4" ("Tab Control 4")) -> ()
          }
        }
      }
      event "Back Stroke step main temperature", "Back SAMPLE TEMPERATURE Step 4", "Back Air TEMPERATURE Step 4": Value Change {
        n654 = event-data() -> ()  [unwired: 1 in, 6 out]
        n655 = stacked-sequence {
          frame #0 {
            n656 = Wait (ms)(milliseconds to wait=u32 1000) -> ()  [unwired: 1 out]
          }
          frame #1 {
            # "CAL;END"
            n657 = local write "Due Write"("CAL;END" ("Command")) -> ()
          }
          frame #2 {
            n658 = Wait (ms)(milliseconds to wait=u32 1000) -> ()  [unwired: 1 out]
          }
          frame #3 {
            # "CAL;END"
            n659 = local write "Due Write"("CAL;END" ("Command")) -> ()
          }
          frame #4 {
            n660 = local write "Main Calibration Tab"(T7."Main" ("Main Calibration Tab")) -> ()
            n661 = local write "Tab Control 4"(T12."Main" ("Tab Control 4")) -> ()
          }
        }
      }
      event "TEMPERATURE STEP  Back 4", "TEMPERATURE STEP 1 Back 3", "TEMPERATURE STEP  Back 3", "TEMPERATURE STEP 1 Back 2": Value Change {
        # "Back Stroke step main temperature"
        n662 = event-data() -> ()  [unwired: 1 in, 6 out]
        n663 = stacked-sequence {
          frame #0 {
            n664 = Wait (ms)(milliseconds to wait=u32 1000) -> ()  [unwired: 1 out]
          }
          frame #1 {
            # "CAL;END"
            n665 = local write "Due Write"("CAL;END" ("Command")) -> ()
          }
          frame #2 {
            n666 = Wait (ms)(milliseconds to wait=u32 1000) -> ()  [unwired: 1 out]
          }
          frame #3 {
            # "CAL;END"
            n667 = local write "Due Write"("CAL;END" ("Command")) -> ()
          }
          frame #4 {
            # "TEMPERATURE STEP  Back 4"
            n668 = local write "Main Calibration Tab"(T7."Temperature" ("Main Calibration Tab")) -> ()
            n669 = local write "Tab Control 4"(T12."Air Step 4" ("Tab Control 4")) -> ()
          }
        }
      }
      event "FF BACK", "FF BACK 2", "FF BACK 3", "FF BACK 4", "FF BACK 5", "FF BACK 6": Value Change {
        n670 = event-data() -> ()  [unwired: 1 in, 6 out]
        n671 = stacked-sequence {
          frame #0 {
            n672 = Wait (ms)(milliseconds to wait=u32 1500) -> ()  [unwired: 1 out]
          }
          frame #1 {
            n673 = local write "Due Write"("VC;0") -> ()
          }
          frame #2 {
            n674 = Wait (ms)(milliseconds to wait=u32 1500) -> ()  [unwired: 1 out]
          }
          frame #3 {
            n675 = local write "Due Write"("VC;0") -> ()
          }
          frame #4 {
            w715 = FALSE
            n676 = local write "FF BACK 6"(w715) -> ()
            n677 = local write "FF BACK 5"(w715) -> ()
            n678 = local write "FF BACK 4"(w715) -> ()
            n679 = local write "FF BACK 3"(w715) -> ()
            n680 = local write "FF BACK 2"(w715) -> ()
            n681 = local write "FF BACK"(w715) -> ()
          }
          frame #5 {
            n682 = local write "Friction Force Tab"(T25."Page 1" ("Friction Force Tab")) -> ()
            n683 = local write "Main Calibration Tab"(T7."Main" ("Main Calibration Tab")) -> ()
          }
        }
      }
      event "FF CONTINUE": Value Change {
        n684 = event-data() -> ()  [unwired: 1 in, 6 out]
        n685 = local write "FF CONTINUE"(FALSE ("FF CONTINUE")) -> ()
        n686 = local write "Friction Force Tab"(T25."Page 2" ("Friction Force Tab")) -> ()
      }
      event "FF CONTINUE 2": Value Change {
        n687 = event-data() -> ()  [unwired: 1 in, 6 out]
        n688 = local write "FF CONTINUE 2"(FALSE ("FF CONTINUE")) -> ()
        n689 = local write "Friction Force Tab"(T25."Page 3" ("Friction Force Tab")) -> ()
      }
      event "FF CONTINUE 3": Value Change {
        n690 = event-data() -> ()  [unwired: 1 in, 6 out]
        n691 = local write "FF CONTINUE 3"(FALSE ("FF CONTINUE")) -> ()
        n692 = local write "Friction Force Tab"(T25."Page 4" ("Friction Force Tab")) -> ()
      }
      event "FF CONTINUE 4": Value Change {
        n693 = event-data() -> ()  [unwired: 1 in, 6 out]
        n694 = local write "FF CONTINUE 4"(FALSE ("FF CONTINUE")) -> ()
        n695 = local write "Friction Force Tab"(T25."Page 5" ("Friction Force Tab")) -> ()
      }
      event "FF CONTINUE 5": Value Change {
        n696 = event-data() -> ()  [unwired: 1 in, 6 out]
        n697 = local write "Friction Force Tab"(T25."Page 6" ("Friction Force Tab")) -> ()
      }
      event "Quit": Value Change {
        n698 = event-data() -> ()  [unwired: 1 in, 6 out]
      }
    }
    n699 = Wait (ms)(milliseconds to wait=u32 100) -> ()  [unwired: 1 out]
  }
  n700 = while {
    stop <- w737 stop-if-true
    n701 = local read "Ambient Temperature"() -> (w735:dbl)
    n702 = local read "Sample Temperature"() -> (w734:dbl)
    n703 = Wait (ms)(milliseconds to wait=u32 200) -> ()  [unwired: 1 out]
    n704 = local write "Sensor value"(w735) -> ()
    n705 = local write "Sensor value"(w735) -> ()
    n706 = local write "Temperature — Live (Set A: 60 °C)"(w735) -> ()
    n707 = local write "Temperature — Live (Set A: 0 °C)"(w735) -> ()
    n708 = local write "Sensor value"(w734) -> ()
    n709 = local write "Sensor value"(w734) -> ()
    n710 = local write "Temperature — Live (Set A: 60 °C)"(w734) -> ()
    n711 = local write "Temperature — Live (Set A: 0 °C)"(w734) -> ()
    n712 = case shown="True" "Save Button" {
      selector: "Save Button" -> [_ w752]
      frame False {
      }
      frame True {
        n713 = Not(x=w752) -> (.not. x?=w751:bool)
        n714 = local read "milliseconds to wait"() -> (w784:u32)
        n715 = local read "max_step_change"() -> (w789:dbl)
        n716 = local read "max_amplitude"() -> (w790:dbl)
        n717 = local read "min_amplitude"() -> (w791:dbl)
        n718 = local read "PIEZO_CAL_FACTOR"() -> (w795:dbl)
        n719 = local write "Save Button"(w751) -> ()
        n720 = local read "startup_cmd"() -> (w792:dbl)
        n721 = local read "NORMAL_FORCE"() -> (w796:dbl)
        n722 = local read "ADC_Resolution"() -> (w794:dbl)
        n723 = local read "calibration values"() -> (w799:dbl[])
        n724 = local read "kd"() -> (w788:dbl)
        n725 = local read "kp"() -> (w786:dbl)
        n726 = local read "dt"() -> (w785:dbl)
        n727 = local read "ki"() -> (w787:dbl)
        n728 = local read "Add up Stroke"() -> (w798:dbl)
        n729 = local read "STROKE FILTER"() -> (w797:i32)
        n730 = local read "VREF"() -> (w793:dbl)
        n731 = Insert Into Array(array=dbl[] [], new element #1=w793, new element #2=w794, new element #3=w795, new element #4=w796) -> (w801:dbl[])  [unwired: 1 in]
        n732 = Insert Into Array(array=dbl[] [], new element #1=w784, new element #2=w785, new element #3=w786, new element #4=w787, new element #5=w788, new element #6=w789, new element #7=w790, new element #8=w791, new element #9=w792) -> (w800:dbl[])  [unwired: 1 in]
        n733 = Array To Spreadsheet String(delimiter (Tab)=";", array=w799, 3:"" ("format string")) -> (spreadsheet string=w803:string)
        n734 = Insert Into Array(array=dbl[] [], new element #1=w797, new element #2=w798) -> (w802:dbl[])  [unwired: 1 in]
        n735 = call "Write Config.vi"("Stroke Calibration"=w803, "STROKE PARAMETERS"=w802, "ADC PARAMETERS"=w801, "PID  PARAMETERS"=w800) -> ("error out"=w782:errorcluster)  [unwired: 7 in]
        n736 = call "Stall Data Flow.vim"("value in"=w782, "milliseconds to wait"=u32 2000) -> ("value out"=w783:errorcluster)  [unwired: 1 out]
        n737 = call "Read Config.vi"("error in (no error)"=w783) -> ("STROKE PARAMETERS"=w780:dbl[], "ADC PARAMETERS"=w779:dbl[], "PID  PARAMETERS"=w778:dbl[], "Stroke Calibration"=w781:string)  [unwired: 6 in, 1 out]
        n738 = Index Array(array=w780) -> (element #1=w763:dbl, element #2=w762:dbl)  [unwired: 2 in]
        n739 = Index Array(array=w779) -> (element #1=w767:dbl, element #2=w766:dbl, element #3=w765:dbl, element #4=w764:dbl)  [unwired: 4 in]
        n740 = Index Array(array=w778) -> (element #1=w776:dbl, element #2=w775:dbl, element #3=w774:dbl, element #4=w773:dbl, element #5=w772:dbl, element #6=w771:dbl, element #7=w770:dbl, element #8=w769:dbl, element #9=w768:dbl)  [unwired: 9 in]
        n741 = Spreadsheet String To Array(delimiter (Tab)=";", format string="", spreadsheet string=w781, array type (2D Dbl)=dbl[] []) -> (array=w777:dbl[])
        n742 = local write "NORMAL_FORCE"(w764) -> ()
        n743 = local write "PIEZO_CAL_FACTOR"(w765) -> ()
        n744 = local write "ADC_Resolution"(w766) -> ()
        n745 = local write "VREF"(w767) -> ()
        n746 = local write "Add up Stroke"(w762) -> ()
        n747 = local write "STROKE FILTER"(w763) -> ()
        n748 = local write "calibration values"(w777) -> ()
        n749 = local write "startup_cmd"(w768) -> ()
        n750 = local write "min_amplitude"(w769) -> ()
        n751 = local write "max_amplitude"(w770) -> ()
        n752 = local write "max_step_change"(w771) -> ()
        n753 = local write "kd"(w772) -> ()
        n754 = local write "ki"(w773) -> ()
        n755 = local write "kp"(w774) -> ()
        n756 = local write "milliseconds to wait"(w776) -> ()
        n757 = local write "dt"(w775) -> ()
      }
    }
    n758 = local read "USER ID"() -> (w732:string)
    n759 = local write "tested by 2"(w732) -> ()
    n760 = local read "run test Calibration"() -> (w731:bool)
    n761 = local read "START TEMP"() -> (w730:bool)
    n762 = And(x=w730, y=w731) -> (x .and. y?=w729:bool)
    n763 = local read "Point 5 - 1.0 mm"() -> (w728:bool)
    n764 = case shown="True" w729 {
      frame False {
        w738 = TRUE ("PAUSE")
        n765 = call "ELAPSED TIMER VI - Calibration.vi"("RESET"=w738, "PAUSE"=w738) -> ()  [unwired: 7 in, 3 out]
      }
      frame True {
        w741 = FALSE ("PAUSE")
        n766 = call "ELAPSED TIMER VI - Calibration.vi"("TARGET"=60.0, "RESET"=w741, "PAUSE"=w741) -> ("ELAPSED INDICATION"=w739:bool)  [unwired: 6 in, 2 out]
        n767 = case shown="True" w739 {
          frame False {
          }
          frame True {
            n768 = stacked-sequence {
              frame #0 {
                n769 = local write "START TEMP"(FALSE ("START TEMP")) -> ()
              }
              frame #1 {
                n770 = Wait (ms)(milliseconds to wait=u32 1500) -> ()  [unwired: 1 out]
              }
              frame #2 {
                n771 = local write "Due Write"("VC;0") -> ()
              }
              frame #3 {
                n772 = Wait (ms)(milliseconds to wait=u32 1500) -> ()  [unwired: 1 out]
              }
              frame #4 {
                n773 = local write "Due Write"("VC;0") -> ()
              }
            }
          }
        }
      }
    }
    n774 = case shown="False" w728 {
      frame False {
        n775 = property on="Accept & Save" class="Bool (strict)"("DisabledEnum"=T19."Disabled" ("Disabled")) -> ()  [unwired: 2 in, 2 out]
        n776 = property on="Tab Control 5" class="TabCtl (strict)"("Value"=enum32{"OK", "NG"}."NG" ("Tab Control 5")) -> ()  [unwired: 2 in, 2 out]
      }
      frame True {
        n777 = property on="Accept & Save" class="Bool (strict)"("DisabledEnum"=T19."Enabled" ("Disabled")) -> ()  [unwired: 2 in, 2 out]
        n778 = property on="Tab Control 5" class="TabCtl (strict)"("Value"=enum32{"OK", "NG"}."OK" ("Tab Control 5")) -> ()  [unwired: 2 in, 2 out]
      }
    }
    n779 = local read "Quit"() -> (w737:bool)
  }
  n780 = while {
    shift-right: [w805] -> _
    shift-left: "Enum - Selector" -> [w806]
    stop <- w807 stop-if-true
    # "Auto Start Logic Loop"
    n781 = case shown="\"Humidity & Temperature On\"" w806 {
      tunnel: [w810 w816 w843 w875 w905 Auto_Start_enum."Exit" ("Enum - Selector") Auto_Start_enum."Init" ("Enum - Selector")] -> w805
      frame "Init", Default {
        n782 = local read "Auto Start Test"() -> (w809:bool)
        n783 = Select(t=Auto_Start_enum."Humidity & Temperature On" ("Enum - Selector"), s=w809, f=Auto_Start_enum."Init") -> (s? t:f=w810:T15)
      }
      frame "Humidity & Temperature On" {
        n784 = stacked-sequence {
          tunnel: [_ _ _ _ _ _ Auto_Start_enum."Reach point" ("Enum - Selector")] -> w813
          frame #0 {
            w818 = T19."Disabled and Grayed Out" ("Disabled")